vi "Dresden R2R Sputter 03.02.2018 IY24.vi"() -> ()   [LabVIEW 2009] (continued)
            n8061 = Boolean Array To Number(Boolean array=w12724) -> (number=w12730:u32)
            n8062 = Mantissa & Exponent(0:w12730) -> (2:w12723:dbl)  [unwired: 1 out]
            n8063 = case shown="0, Default" w12723 {
              tunnel: [u16 0 ("Starting Address") u16 1184 ("Starting Address") u16 1185 ("Starting Address") u16 1186 ("Starting Address") u16 1187 ("Starting Address")] -> w12720
              tunnel: [u16 0 ("Ao_1_3") "Ch4_Ao_1_0 4" "Ch4_Ao_1_1 4" "Ch4_Ao_1_2 4" "Ch4_Ao_1_3 4"] -> w12722
              frame #0 {
              }
              frame #1 {
              }
              frame #2 {
              }
              frame #3 {
              }
              frame #4 {
              }
            }
            n8064 = Build Array(w12722) -> (w12721:u16[])
            n8065 = call-poly <vilib>:"MB Serial Master Query (poly).vi"("VISA resource name"=w12719, "Starting Address"=w12720, "Registers"=w12721, "error in"=w12718, "Serial Parameters"=T39 {"Mode"=enum."RTU", "Slave Address"=6}) -> ("VISA resource name out"=w12732:refnum<visa-resource-name>, "error out"=w12731:errorcluster)  [unwired: 1 in, 12 out]
          }
          frame #7 {
            n8066 = Wait (ms)(milliseconds to wait=w12744) -> ()  [unwired: 1 out]
          }
        }
      }
      frame #1 {
        n8067 = local read "Fail_moxa4_digital3"() -> (w12747:bool)
        n8068 = local read "Fail_moxa4_digital4"() -> (w12746:bool)
        n8069 = local read "Fail_moxa4_digital1"() -> (w12745:bool)
        n8070 = local read "Fail_moxa4_digital2"() -> (w12748:bool)
        n8071 = case shown="True" w12748 {
          frame #0 {
            n8072 = local read "Ch4_Trns_gv_bp_do"() -> (w12767:bool)
            n8073 = local read "Ch4_Trns_gv_bp_di"() -> (w12766:bool)
            n8074 = Exclusive Or(1:w12767, 2:w12766) -> (0:w12765:bool)
            n8075 = feedback #213() -> (w12764:bool)  [unwired: 1 in]
            n8076 = case shown="True" w12765 {
              tunnel: [TRUE FALSE] -> w12763
              tunnel: w12764 -> [_ w12787]
              tunnel: [FALSE w12784] -> w12762
              frame #0 {
              }
              frame #1 {
                n8077 = call "Elapsed Time117"("Reset"=w12787) -> ("Elapsed Time (s)"=w12786:dbl)  [unwired: 11 in, 7 out]
                n8078 = Greater?(x=w12786, y=5.0) -> (0:w12784:bool)
              }
            }
            n8079 = local write "Trns_gv_bp_ch4_fail_top"(w12762) -> ()
            n8080 = local write "Trns_gv_bp_fail_ch4_front"(w12762) -> ()
            n8081 = local write "Ch4_Trns_gv_bp_fail"(w12762) -> ()
            n8082 = local read "Ch4_Sov_Ar_do"() -> (w12761:bool)
            n8083 = local read "Ch4_Sov_Ar_di"() -> (w12760:bool)
            n8084 = Exclusive Or(1:w12761, 2:w12760) -> (0:w12759:bool)
            n8085 = feedback #214() -> (w12758:bool)  [unwired: 1 in]
            n8086 = case shown="True" w12759 {
              tunnel: [TRUE FALSE] -> w12757
              tunnel: w12758 -> [_ w12780]
              tunnel: [FALSE w12777] -> w12756
              frame #0 {
              }
              frame #1 {
                n8087 = call "Elapsed Time110"("Reset"=w12780) -> ("Elapsed Time (s)"=w12779:dbl)  [unwired: 11 in, 7 out]
                n8088 = Greater?(x=w12779, y=5.0) -> (0:w12777:bool)
              }
            }
            n8089 = local write "ch4_sov_Ar_fail_top"(w12756) -> ()
            n8090 = local read "Ch4_Cst_fix_down_di"() -> (w12752:bool)
            n8091 = local read "Ch4_Cst_fix_do"() -> (w12751:bool)
            n8092 = Exclusive Or(1:w12752, 2:w12751) -> (0:w12755:bool)
            n8093 = feedback #215() -> (w12753:bool)  [unwired: 1 in]
            n8094 = case shown="True" w12755 {
              tunnel: [TRUE FALSE] -> w12754
              tunnel: w12753 -> [_ w12773]
              tunnel: [FALSE w12770] -> w12750
              frame #0 {
              }
              frame #1 {
                n8095 = call "Elapsed Time189"("Reset"=w12773) -> ("Elapsed Time (s)"=w12772:dbl)  [unwired: 11 in, 7 out]
                n8096 = Greater?(x=w12772, y=60.0) -> (0:w12770:bool)
              }
            }
            n8097 = local write "chamber 4 top piston failed"(w12750) -> ()
          }
          frame #1 {
            w12789 = TRUE ("Ch_bv_fail(ch4)L")
            n8098 = local write "Trns_gv_bp_ch4_fail_top"(w12789) -> ()
            n8099 = local write "Trns_gv_bp_fail_ch4_front"(w12789) -> ()
            n8100 = local write "Ch4_Trns_gv_bp_fail"(w12789) -> ()
            n8101 = local write "chamber 4 top piston failed"(w12789) -> ()
            n8102 = local write "ch4_sov_Ar_fail_top"(w12789) -> ()
          }
        }
        n8103 = case shown="True" w12745 {
          frame #0 {
            w12790 = TRUE
            n8104 = local write "ch4_atm_fail_top"(w12790) -> ()
            n8105 = local write "Ch4_Ch_vbv_fail"(w12790) -> ()
            n8106 = local write "Ch4_Ch_atm_fail"(w12790) -> ()
            n8107 = local write "ch1_bg_bv_fail_top"(w12790) -> ()
            n8108 = local write "Ch4_Bg_bv_fail"(w12790) -> ()
            n8109 = local write "Ch4_Tp_bv_fail"(w12790) -> ()
            n8110 = local write "Ch4_Mp_fail"(w12790) -> ()
            n8111 = local write "ch4_bg_bv_fail_top"(w12790) -> ()
            n8112 = local write "Ch4_Ch_cc_fail"(w12790) -> ()
            n8113 = local write "Ch4_Pl_vbv_fail"(w12790) -> ()
            n8114 = local write "Ch4_Pl_atm_fail"(w12790) -> ()
            n8115 = local write "ch4_cc_fail_top"(w12790) -> ()
          }
          frame #1 {
            n8116 = local read "Ch4_Mp_do"() -> (w12807:bool)
            n8117 = local read "Ch4_Mp_di"() -> (w12808:bool)
            n8118 = Exclusive Or(1:w12807, 2:w12808) -> (0:w12824:bool)
            n8119 = feedback #216() -> (w12825:bool)  [unwired: 1 in]
            n8120 = case shown="True" w12824 {
              tunnel: [TRUE FALSE] -> w12826
              tunnel: w12825 -> [_ w12867]
              tunnel: [FALSE w12864] -> w12806
              frame #0 {
              }
              frame #1 {
                n8121 = call "Elapsed Time122"("Reset"=w12867) -> ("Elapsed Time (s)"=w12866:dbl)  [unwired: 11 in, 7 out]
                n8122 = Greater?(x=w12866, y=5.0) -> (0:w12864:bool)
              }
            }
            n8123 = local write "Ch4_Mp_fail"(w12806) -> ()
            n8124 = local read "Ch4_Tp_bv_do"() -> (w12804:bool)
            n8125 = local read "Ch4_Tp_bv_di"() -> (w12805:bool)
            n8126 = Exclusive Or(1:w12804, 2:w12805) -> (0:w12823:bool)
            n8127 = feedback #217() -> (w12822:bool)  [unwired: 1 in]
            n8128 = case shown="True" w12823 {
              tunnel: [TRUE FALSE] -> w12821
              tunnel: w12822 -> [_ w12860]
              tunnel: [FALSE w12857] -> w12803
              frame #0 {
              }
              frame #1 {
                n8129 = call "Elapsed Time123"("Reset"=w12860) -> ("Elapsed Time (s)"=w12859:dbl)  [unwired: 11 in, 7 out]
                n8130 = Greater?(x=w12859, y=5.0) -> (0:w12857:bool)
              }
            }
            n8131 = local write "Ch4_Tp_bv_fail"(w12803) -> ()
            n8132 = local read "Ch4_Bg_bv_di"() -> (w12802:bool)
            n8133 = local read "Ch4_Bg_bv_do"() -> (w12801:bool)
            n8134 = Exclusive Or(1:w12801, 2:w12802) -> (0:w12818:bool)
            n8135 = feedback #218() -> (w12819:bool)  [unwired: 1 in]
            n8136 = case shown="True" w12818 {
              tunnel: [TRUE FALSE] -> w12820
              tunnel: w12819 -> [_ w12853]
              tunnel: [FALSE w12850] -> w12792
              frame #0 {
              }
              frame #1 {
                n8137 = call "Elapsed Time124"("Reset"=w12853) -> ("Elapsed Time (s)"=w12852:dbl)  [unwired: 11 in, 7 out]
                n8138 = Greater?(x=w12852, y=5.0) -> (0:w12850:bool)
              }
            }
            n8139 = local write "ch4_bg_bv_fail_top"(w12792) -> ()
            n8140 = local write "Ch4_Bg_bv_fail"(w12792) -> ()
            n8141 = local read "Ch4_Ch_vbv_do"() -> (w12799:bool)
            n8142 = local read "Ch4_Ch_vbv_di"() -> (w12800:bool)
            n8143 = Exclusive Or(1:w12799, 2:w12800) -> (0:w12817:bool)
            n8144 = feedback #219() -> (w12816:bool)  [unwired: 1 in]
            n8145 = case shown="True" w12817 {
              tunnel: [TRUE FALSE] -> w12815
              tunnel: w12816 -> [_ w12846]
              tunnel: [FALSE w12843] -> w12793
              frame #0 {
              }
              frame #1 {
                n8146 = call "Elapsed Time125"("Reset"=w12846) -> ("Elapsed Time (s)"=w12845:dbl)  [unwired: 11 in, 7 out]
                n8147 = Greater?(x=w12845, y=5.0) -> (0:w12843:bool)
              }
            }
            n8148 = local write "Ch4_Ch_vbv_fail"(w12793) -> ()
            n8149 = local read "Ch4_Pl_vbv_do"() -> (w12796:bool)
            n8150 = local read "Ch4_Pl_vbv_di"() -> (w12797:bool)
            n8151 = Exclusive Or(1:w12796, 2:w12797) -> (0:w12814:bool)
            n8152 = feedback #220() -> (w12813:bool)  [unwired: 1 in]
            n8153 = case shown="True" w12814 {
              tunnel: [TRUE FALSE] -> w12812
              tunnel: w12813 -> [_ w12839]
              tunnel: [FALSE w12836] -> w12798
              frame #0 {
              }
              frame #1 {
                n8154 = call "Elapsed Time127"("Reset"=w12839) -> ("Elapsed Time (s)"=w12838:dbl)  [unwired: 11 in, 7 out]
                n8155 = Greater?(x=w12838, y=5.0) -> (0:w12836:bool)
              }
            }
            n8156 = local write "Ch4_Pl_vbv_fail"(w12798) -> ()
            n8157 = local read "Ch4_Cc_on_off_di"() -> (w12795:bool)
            n8158 = local read "Ch4_Cc_on_off_do"() -> (w12794:bool)
            n8159 = feedback #221() -> (w12810:bool)  [unwired: 1 in]
            n8160 = Exclusive Or(1:w12794, 2:w12795) -> (0:w12811:bool)
            n8161 = case shown="True" w12811 {
              tunnel: [TRUE FALSE] -> w12809
              tunnel: w12810 -> [_ w12832]
              tunnel: [FALSE w12829] -> w12791
              frame #0 {
              }
              frame #1 {
                n8162 = call "Elapsed Time129"("Reset"=w12832) -> ("Elapsed Time (s)"=w12831:dbl)  [unwired: 11 in, 7 out]
                n8163 = Greater?(x=w12831, y=5.0) -> (0:w12829:bool)
              }
            }
            n8164 = local write "ch4_cc_fail_top"(w12791) -> ()
          }
        }
        n8165 = case shown="True" w12747 {
          frame #0 {
          }
          frame #1 {
          }
        }
        n8166 = case shown="False" w12746 {
          frame #0 {
          }
          frame #1 {
            n8167 = local write "Ch4_Trns_gv_bp_fail"(TRUE ("Ch_bv_fail(ch4)L")) -> ()
          }
        }
      }
    }
    n8168 = Wait Until Next ms Multiple(millisecond multiple=u32 300) -> ()  [unwired: 1 out]
  }
  n8169 = while {
    tunnel: w760 -> [w12875]
    tunnel: [w12874] -> w744
    tunnel: [w12873] -> w759
    tunnel: w761 -> [w12872]
    tunnel: "milliseconds to wait 4" -> [w12870]
    stop <- FALSE stop-if-true
    n8170 = Wait Until Next ms Multiple(millisecond multiple=u32 300) -> ()  [unwired: 1 out]
    n8171 = stacked-sequence {
      tunnel: w12875 -> [w12880 _]
      tunnel: [w12879 _] -> w12874
      tunnel: [w12877 _] -> w12873
      tunnel: w12872 -> [w12878 _]
      tunnel: w12870 -> [w12876 _]
      frame #0 {
        n8172 = stacked-sequence {
          tunnel: w12878 -> [w12903 _ _ _ _ _ _ _ _ _]
          tunnel: w12880 -> [w12902 _ _ _ _ _ _ _ _ _]
          tunnel: [_ _ _ _ _ _ _ _ w13238 _] -> w12879
          tunnel: [_ _ _ _ _ _ _ _ w13237 _] -> w12877
          tunnel: w12876 -> [_ w12973 _ w12993 _ w13048 _ w13224 _ w13257]
          frame #0 {
            # "Digital I/O & Analog \nOutput Part"
            n8173 = call-poly <vilib>:"MB Serial Master Query (poly).vi"("VISA resource name"=w12903, "Starting Address"=u16 0, "Quantity"=u16 8, "error in"=w12902, "Serial Parameters"=T39 {"Mode"=enum."RTU", "Slave Address"=1}) -> ("VISA resource name out"=w12901:refnum<visa-resource-name>, "Discrete Inputs"=w12962:bool[], "error out"=w12900:errorcluster)  [unwired: 1 in, 11 out]
            n8174 = Index Array(array=w12962, index=6) -> (element=w12957:bool)
            "Ch3_Pl_atm_di" <- w12957
            n8175 = Index Array(array=w12962, index=7) -> (element=w12886:bool)
            "Ch3_Cc_on_off_di" <- w12886
            n8176 = Index Array(array=w12962, index=5) -> (element=w12891:bool)
            "Ch3_Pl_vbv_di" <- w12891
            n8177 = Index Array(array=w12962, index=0) -> (element=w12960:bool)
            "Ch3_Mp_di" <- w12960
            n8178 = Index Array(array=w12962, index=1) -> (element=w12959:bool)
            "Ch3_Tp_bv_di" <- w12959
            n8179 = Index Array(array=w12962, index=2) -> (element=w12888:bool)
            "Ch3_Bg_bv_di" <- w12888
            n8180 = Index Array(array=w12962, index=3) -> (element=w12958:bool)
            "Ch3_Ch_vbv_di" <- w12958
            n8181 = Index Array(array=w12962, index=4) -> (element=w12887:bool)
            "Ch3_Ch_atm_di" <- w12887
            n8182 = local write "Ch3_Mp_on"(w12960) -> ()
            n8183 = local write "Ch3_Tp_bv_on"(w12959) -> ()
            n8184 = local write "ch3_bg_bv_on_top"(w12888) -> ()
            n8185 = local write "Ch3_Bg_bv_on"(w12888) -> ()
            n8186 = local write "Ch3_Ch_vbv_on"(w12958) -> ()
            n8187 = local write "ch3_atm_on_top"(w12887) -> ()
            n8188 = local write "Ch3_Ch_atm_on"(w12887) -> ()
            n8189 = local write "Ch3_Pl_vbv_on"(w12891) -> ()
            n8190 = local write "Ch3_Pl_atm_on"(w12957) -> ()
            n8191 = local write "Ch3_Ch_cc_on"(w12886) -> ()
            n8192 = local write "ch3_cc_on_top"(w12886) -> ()
            n8193 = local read "Load_dido"() -> (w12890:bool)
            n8194 = case shown="True" w12890 {
              frame #0 {
              }
              frame #1 {
                n8195 = Wait (ms)(milliseconds to wait=u32 2000) -> ()  [unwired: 1 out]
              }
            }
            n8196 = call-poly <vilib>:"MB Serial Master Query (poly).vi"("VISA resource name"=w12901, "Starting Address"=u16 0, "Quantity"=u16 8, "error in"=w12900, "Serial Parameters"=T39 {"Mode"=enum."RTU", "Slave Address"=2}) -> ("VISA resource name out"=w12899:refnum<visa-resource-name>, "Discrete Inputs"=w12947:bool[], "error out"=w12898:errorcluster)  [unwired: 1 in, 11 out]
            n8197 = Index Array(array=w12947, index=2) -> (element=→"Ch3_Trns_gv_close_di":bool)
            n8198 = Index Array(array=w12947, index=0) -> (element=w12889:bool)
            "Ch3_Sov_Ar_di" <- w12889
            n8199 = Index Array(array=w12947, index=1) -> (element=w12883:bool)
            "Ch3_Trns_gv_open_di" <- w12883
            n8200 = Index Array(array=w12947, index=5) -> (element=w12884:bool)
            "Ch3_Cst_fix_down_di" <- w12884
            n8201 = Index Array(array=w12947, index=6) -> (element=→"Ch3_Pet_cool_up_di":bool)
            n8202 = Index Array(array=w12947, index=7) -> (element=→"Ch3_Pet_cool_down_di":bool)
            n8203 = Index Array(array=w12947, index=3) -> (element=w12881:bool)
            "Ch3_Trns_gv_bp_di" <- w12881
            n8204 = Index Array(array=w12947, index=4) -> (element=→"Ch3_Cst_fix_up_di":bool)
            n8205 = local write "Ch3_trns_gv_bp_on_front"(w12881) -> ()
            n8206 = local write "gv front_open_ch3_4"(w12883) -> ()
            n8207 = local write "Trns_gv_3_4_on"(w12883) -> ()
            n8208 = local write "gv top open_ch3_4"(w12883) -> ()
            n8209 = local write "gv front open ch4_3"(w12883) -> ()
            n8210 = local write "gv top open ch_4_3"(w12883) -> ()
            n8211 = local write "Ch3_Trns_gv_bp_on"(w12881) -> ()
            n8212 = local write "ch3_sov_Ar_on_top"(w12889) -> ()
            n8213 = local write "chamber 3 top piston open"(w12884) -> ()
            n8214 = local write "ch3_trns_gv_bp_on_top"(w12881) -> ()
            n8215 = call-poly <vilib>:"MB Serial Master Query (poly).vi"("VISA resource name"=w12899, "Starting Address"=u16 0, "Quantity"=u16 8, "error in"=w12898, "Serial Parameters"=T39 {"Mode"=enum."RTU", "Slave Address"=3}) -> ("VISA resource name out"=w12897:refnum<visa-resource-name>, "Discrete Inputs"=w12907:bool[], "error out"=w12896:errorcluster)  [unwired: 1 in, 11 out]
            n8216 = Index Array(array=w12907, index=5) -> (element=→"Ch3_SRV2_counter_di":bool)
            n8217 = Index Array(array=w12907, index=6) -> (element=→"Ch3_WFS_di":bool)
            n8218 = Index Array(array=w12907, index=7) -> (element=w12882:bool)
            "Ch3_Trns_gv_bp2_di" <- w12882
            n8219 = Index Array(array=w12907, index=0) -> (element=→"Ch3_SRV1_PIST For_di":bool)
            n8220 = Index Array(array=w12907, index=1) -> (element=→"Ch3_SRV1_PIST_Back_di":bool)
            n8221 = Index Array(array=w12907, index=2) -> (element=→"Ch3_SRV_start_stop_di":bool)
            n8222 = Index Array(array=w12907, index=3) -> (element=→"Ch3_SRV_left_direction_di":bool)
            n8223 = Index Array(array=w12907, index=4) -> (element=→"Ch3_SRV1_counter_di":bool)
            n8224 = local write "Ch3_Trns_gv_bp2_on"(w12882) -> ()
            n8225 = local write "ch3_trns_gv_bp2_on_top"(w12882) -> ()
            n8226 = local write "Ch3_trns_gv_bp2_on_front"(w12882) -> ()
            n8227 = call-poly <vilib>:"MB Serial Master Query (poly).vi"("VISA resource name"=w12897, "Starting Address"=u16 0, "Quantity"=u16 8, "error in"=w12896, "Serial Parameters"=T39 {"Mode"=enum."RTU", "Slave Address"=4}) -> ("VISA resource name out"=w12895:refnum<visa-resource-name>, "Discrete Inputs"=w12931:bool[], "error out"=w12894:errorcluster)  [unwired: 1 in, 11 out]
            n8228 = Index Array(array=w12931, index=5) -> (element=→"Ch3_Right_slow_di":bool)
            n8229 = Index Array(array=w12931, index=6) -> (element=→"Ch3_Left_slow_di":bool)
            n8230 = Index Array(array=w12931, index=7) -> (element=→"Ch3_Left_limit_di":bool)
            n8231 = Index Array(array=w12931, index=0) -> (element=→"Ch3_Air_press_di":bool)
            n8232 = Index Array(array=w12931, index=1) -> (element=→"Ch3_Ds_di":bool)
            n8233 = Index Array(array=w12931, index=2) -> (element=→"Ch3_TGV_control_di":bool)
            n8234 = Index Array(array=w12931, index=3) -> (element=→"Ch3_Trns_interlock_di":bool)
            n8235 = Index Array(array=w12931, index=4) -> (element=→"Ch3_Right_limit_di":bool)
          }
          frame #1 {
            n8236 = Wait (ms)(milliseconds to wait=w12973) -> ()  [unwired: 1 out]
          }
          frame #2 {
            n8237 = local read "Load_dido"() -> (w12974:bool)
            n8238 = case shown="True" w12974 {
              frame #0 {
              }
              frame #1 {
                n8239 = while {
                  stop <- w12986 stop-if-true
                  n8240 = local read "Ch3_Mp_di"() -> (w12992:bool)
                  n8241 = local read "Ch3_Tp_bv_di"() -> (w12991:bool)
                  n8242 = local read "Ch3_Bg_bv_di"() -> (w12990:bool)
                  n8243 = local read "Ch3_Ch_vbv_di"() -> (w12989:bool)
                  n8244 = local read "Ch3_Pl_vbv_di"() -> (w12988:bool)
                  n8245 = local read "Ch3_Cc_on_off_di"() -> (w12987:bool)
                  n8246 = local write "Ch3_Mp_do"(w12992) -> ()
                  n8247 = local write "Ch3_Tp_bv_do"(w12991) -> ()
                  n8248 = local write "Ch3_Bg_bv_do"(w12990) -> ()
                  n8249 = local write "Ch3_Ch_vbv_do"(w12989) -> ()
                  n8250 = local write "Ch3_Pl_vbv_do"(w12988) -> ()
                  n8251 = local write "Ch3_Cc_on_off_do"(w12987) -> ()
                  n8252 = local read "Ch3_Trns_gv_bp2_di"() -> (w12982:bool)
                  n8253 = Wait Until Next ms Multiple(millisecond multiple=u32 300) -> ()  [unwired: 1 out]
                  n8254 = local read "Ch3_WFS_di"() -> (w12983:bool)
                  n8255 = local write "Ch3_WFC_do"(w12983) -> ()
                  n8256 = local write "Ch3_Trns_gv_bp2_do"(w12982) -> ()
                  n8257 = local read "Ch3_Cst_fix_down_di"() -> (w12977:bool)
                  n8258 = local read "Ch3_Sov_Ar_di"() -> (w12981:bool)
                  n8259 = local read "Ch3_Trns_gv_open_di"() -> (w12980:bool)
                  n8260 = local read "Ch3_Trns_gv_close_di"() -> (w12979:bool)
                  n8261 = local read "Ch3_Pet_cool_up_di"() -> (w12976:bool)
                  n8262 = local read "Ch3_Pet_cool_down_di"() -> (w12975:bool)
                  n8263 = local read "Ch3_Trns_gv_bp_di"() -> (w12978:bool)
                  n8264 = local write "Ch3_Sov_Ar_do"(w12981) -> ()
                  n8265 = local write "Ch3_Trns_gv_open_do"(w12980) -> ()
                  n8266 = local write "Ch3_Trns_gv_close_do"(w12979) -> ()
                  n8267 = local write "Ch3_Pet_cool_up_do"(w12976) -> ()
                  n8268 = local write "Ch3_Pet_cool_down_do"(w12975) -> ()
                  n8269 = local write "Ch3_Trns_gv_bp_do"(w12978) -> ()
                  n8270 = local write "Ch3_Cst_fix_do"(w12977) -> ()
                  n8271 = local read "Load_dido"() -> (w12985:bool)
                  n8272 = Not(x=w12985) -> (.not. x?=w12986:bool)
                }
              }
            }
          }
          frame #3 {
            n8273 = Wait (ms)(milliseconds to wait=w12993) -> ()  [unwired: 1 out]
          }
          frame #4 {
            n8274 = Build Array("Ch3_Mp_do", "Ch3_Tp_bv_do", "Ch3_Bg_bv_do", "Ch3_Ch_vbv_do", "Ch3_Ch_atm_do", "Ch3_Pl_vbv_do", "Ch3_Pl_atm_do", "Ch3_Cc_on_off_do") -> (w13018:bool[])
            n8275 = call-poly <vilib>:"MB Serial Master Query (poly).vi"("VISA resource name"=w13005, "Starting Address"=u16 320, "Coils"=w13018, "error in"=w13004, "Serial Parameters"=T39 {"Mode"=enum."RTU", "Slave Address"=1}) -> ("VISA resource name out"=w13003:refnum<visa-resource-name>, "error out"=w13002:errorcluster)  [unwired: 1 in, 12 out]
            n8276 = Build Array("Ch3_Sov_Ar_do", "Ch3_Trns_gv_open_do", "Ch3_Trns_gv_close_do", "Ch3_Trns_gv_bp_do", "Ch3_Cst_fix_do", "Ch3_2_5_do", "Ch3_Pet_cool_up_do", "Ch3_Pet_cool_down_do") -> (w13028:bool[])
            n8277 = call-poly <vilib>:"MB Serial Master Query (poly).vi"("VISA resource name"=w13003, "Starting Address"=u16 320, "Coils"=w13028, "error in"=w13002, "Serial Parameters"=T39 {"Mode"=enum."RTU", "Slave Address"=2}) -> ("VISA resource name out"=w13001:refnum<visa-resource-name>, "error out"=w13000:errorcluster)  [unwired: 1 in, 12 out]
            n8278 = Build Array("Ch3_SRV1_PIST For_do", "Ch3_SRV1_PIST_Back_do", "Ch3_SRV_start_stop_do", "Ch3_SRV_counterclockwise_direction_do", "Ch3_Do_3_4", "Ch3_Do_3_5", "Ch3_WFC_do", "Ch3_Trns_gv_bp2_do") -> (w13036:bool[])
            n8279 = call-poly <vilib>:"MB Serial Master Query (poly).vi"("VISA resource name"=w13001, "Starting Address"=u16 320, "Coils"=w13036, "error in"=w13000, "Serial Parameters"=T39 {"Mode"=enum."RTU", "Slave Address"=3}) -> ("VISA resource name out"=w12998:refnum<visa-resource-name>, "error out"=w12999:errorcluster)  [unwired: 1 in, 12 out]
            n8280 = Build Array("Ch3_4_0_do", "Ch3_4_1_do", "Ch3_TGV_control_do", "Ch3_4_3_do", "Ch3_4_4_do", "Ch3_Do_4_5_do", "Ch3_Do_4_6_do", "Ch3_Do_4_6_do") -> (w13038:bool[])
            n8281 = call-poly <vilib>:"MB Serial Master Query (poly).vi"("VISA resource name"=w12998, "Starting Address"=u16 320, "Coils"=w13038, "error in"=w12999, "Serial Parameters"=T39 {"Mode"=enum."RTU", "Slave Address"=4}) -> ("VISA resource name out"=w12997:refnum<visa-resource-name>, "error out"=w12996:errorcluster)  [unwired: 1 in, 12 out]
          }
          frame #5 {
            n8282 = Wait (ms)(milliseconds to wait=w13048) -> ()  [unwired: 1 out]
          }
          frame #6 {
            n8283 = local read "1bit="() -> (w13059:dbl)
            n8284 = local read "1bit="() -> (w13061:dbl)
            n8285 = local read "1bit="() -> (w13053:dbl)
            n8286 = call-poly <vilib>:"MB Serial Master Query (poly).vi"("VISA resource name"=w13057, "Starting Address"=u16 704, "Quantity"=u16 8, "error in"=w13055, "Serial Parameters"=T39 {"Mode"=enum."RTU", "Slave Address"=5}) -> ("VISA resource name out"=w13056:refnum<visa-resource-name>, "Input Registers"=w13069:u16[], "error out"=w13054:errorcluster)  [unwired: 1 in, 11 out]
            n8287 = Index Array(array=w13069, index=5) -> (element=→"Ch1_Ai_1_5 3":u16)
            n8288 = Index Array(array=w13069, index=6) -> (element=→"Ch1_Ai_1_6 3":u16)
            n8289 = Index Array(array=w13069, index=7) -> (element=→"Ch1_Ai_1_7 3":u16)
            n8290 = Index Array(array=w13069, index=0) -> (element=w13063:u16)
            "Ch3_Ai_PL_PG" <- w13063
            n8291 = Index Array(array=w13069, index=1) -> (element=w13049:u16)
            "Ch3_Ai_CH_PG" <- w13049
            n8292 = Multiply(x=w13061, y=w13049) -> (x*y=w13060:dbl)
            n8293 = stacked-sequence {
              tunnel: w13060 -> [w13161]
              frame #0 {
                # "CH-PG 0-10 Volt okuma"
                n8294 = feedback #222() -> (w13172:dbl)  [unwired: 1 in]
                n8295 = feedback #223() -> (w13170:dbl)  [unwired: 1 in]
                n8296 = feedback #224() -> (w13169:dbl)  [unwired: 1 in]
                n8297 = feedback #225() -> (w13168:dbl)  [unwired: 1 in]
                n8298 = feedback #226() -> (w13167:dbl)  [unwired: 1 in]
                n8299 = feedback #227() -> (w13166:dbl)  [unwired: 1 in]
                n8300 = feedback #228() -> (w13165:dbl)  [unwired: 1 in]
                n8301 = feedback #229() -> (w13163:dbl)  [unwired: 1 in]
                n8302 = feedback #230() -> (w13164:dbl)  [unwired: 1 in]
                n8303 = Compound Arithmetic op=ADD(w13161, w13172, w13170, w13169, w13168, w13167, w13166, w13165, w13163, w13164) -> (w13171:dbl)
                n8304 = local read "Ch_pg_volt_instantaneos_ch3"() -> (w13155:u16)
                n8305 = Divide(x=w13171, y=u16 10) -> (x/y=w13156:dbl)
                "Ch_pg_volt_ch3" <- w13156
                n8306 = Greater Or Equal?(x=w13155, y=u16 1) -> (x >= y?=w13154:bool)
                n8307 = feedback #231() -> (w13159:bool)  [unwired: 1 in]
                n8308 = case shown="True" w13154 {
                  tunnel: w13156 -> [_ w13184]
                  tunnel: [FALSE TRUE] -> w13158
                  tunnel: w13159 -> [w13175 _]
                  tunnel: [w13174 FALSE ("Bg_gui")] -> w13160
                  frame #0 {
                    n8309 = local write "Ch3_Ch_pg_on"(FALSE ("Bg_gui")) -> ()
                    n8310 = call "Elapsed Time143"("Reset"=w13175) -> ("Elapsed Time (s)"=w13178:dbl)  [unwired: 11 in, 7 out]
                    n8311 = Greater Or Equal?(x=w13178, y=3.0) -> (x >= y?=w13174:bool)
                  }
                  frame #1 {
                    n8312 = Subtract(x=w13184, y=5.625) -> (x-y=w13186:dbl)
                    n8313 = Power Of 10(x=w13186) -> (10^x=w13185:dbl)
                    n8314 = In Range and Coerce(upper limit=760.0, x=w13185, lower limit=0.000375) -> (coerced(x)=→"Ch_pg_press_ch3" →"Ch_pg_press_ch3_gui":dbl)  [unwired: 1 out]
                    n8315 = local write "Ch3_Ch_pg_on"(TRUE ("Bg_gui")) -> ()
                  }
                }
                n8316 = local write "Ch3_Ch_pg_fail"(w13160) -> ()
                "Ch_pg_volt_instantaneos_ch3" <- w13161
              }
            }
            n8317 = Index Array(array=w13069, index=2) -> (element=w13050:u16)
            "Ch3_Ai_CH-CC" <- w13050
            n8318 = Multiply(x=w13059, y=w13050) -> (x*y=w13058:dbl)
            n8319 = stacked-sequence {
              tunnel: w13058 -> [w13106]
              frame #0 {
                # "CH-CC 0-10 Volt okuma"
                n8320 = feedback #232() -> (w13115:dbl)  [unwired: 1 in]
                n8321 = feedback #233() -> (w13116:dbl)  [unwired: 1 in]
                n8322 = feedback #234() -> (w13117:dbl)  [unwired: 1 in]
                n8323 = feedback #235() -> (w13118:dbl)  [unwired: 1 in]
                n8324 = feedback #236() -> (w13119:dbl)  [unwired: 1 in]
                n8325 = feedback #237() -> (w13120:dbl)  [unwired: 1 in]
                n8326 = feedback #238() -> (w13121:dbl)  [unwired: 1 in]
                n8327 = feedback #239() -> (w13133:dbl)  [unwired: 1 in]
                n8328 = feedback #240() -> (w13122:dbl)  [unwired: 1 in]
                n8329 = feedback #241() -> (w13123:dbl)  [unwired: 1 in]
                n8330 = feedback #242() -> (w13124:dbl)  [unwired: 1 in]
                n8331 = feedback #243() -> (w13125:dbl)  [unwired: 1 in]
                n8332 = feedback #244() -> (w13126:dbl)  [unwired: 1 in]
                n8333 = feedback #245() -> (w13127:dbl)  [unwired: 1 in]
                n8334 = feedback #246() -> (w13128:dbl)  [unwired: 1 in]
                n8335 = feedback #247() -> (w13129:dbl)  [unwired: 1 in]
                n8336 = feedback #248() -> (w13130:dbl)  [unwired: 1 in]
                n8337 = feedback #249() -> (w13131:dbl)  [unwired: 1 in]
                n8338 = feedback #250() -> (w13132:dbl)  [unwired: 1 in]
                n8339 = Compound Arithmetic op=ADD(w13106, w13115, w13116, w13117, w13118, w13119, w13120, w13121, w13133, w13122, w13123, w13124, w13125, w13126, w13127, w13128, w13129, w13130, w13131, w13132) -> (w13114:dbl)
                n8340 = Divide(x=w13114, y=u16 20) -> (x/y=w13110:dbl)
                "Ch_CC_volt ch3" <- w13110
                n8341 = feedback #251() -> (w13107:bool)  [unwired: 1 in]
                n8342 = Greater?(x=w13110, y=1.0) -> (0:w13111:bool)
                n8343 = case shown="True" w13111 {
                  tunnel: w13110 -> [_ w13150]
                  tunnel: [w13141 FALSE] -> w13109
                  tunnel: [FALSE ("Ch_cc_on(ch1)") TRUE] -> w13108
                  tunnel: w13107 -> [_ _]
                  frame #0 {
                    n8344 = local read "Ch3_Cc_on_off_di"() -> (w13135:bool)
                    n8345 = call "Elapsed Time87"() -> ("Elapsed Time (s)"=w13144:dbl)  [unwired: 12 in, 7 out]
                    n8346 = Not(x=w13135) -> (.not. x?=w13138:bool)
                    n8347 = Greater Or Equal?(x=w13144, y=3.0) -> (x >= y?=w13143:bool)
                    n8348 = call "Elapsed Time88"("Reset"=w13138) -> ("Elapsed Time (s)"=w13140:dbl)  [unwired: 11 in, 7 out]
                    n8349 = local write "Ch3_Ch_cc_on"(FALSE ("Ch_cc_on(ch1)")) -> ()
                    n8350 = Greater Or Equal?(x=w13140, y=3.0) -> (x >= y?=w13137:bool)
                    n8351 = And(x=w13143, y=w13137) -> (x .and. y?=w13141:bool)
                  }
                  frame #1 {
                    n8352 = Subtract(x=w13150, y=10.625) -> (x-y=w13147:dbl)
                    n8353 = Power Of 10(x=w13147) -> (10^x=w13146:dbl)
                    n8354 = In Range and Coerce(upper limit=0.0075, x=w13146, lower limit=1.5e-09) -> (coerced(x)=→"Ch_CC_press_ch3" →"Ch_CC_press_ch3 2":dbl)  [unwired: 1 out]
                  }
                }
                n8355 = local write "Ch3_Ch_cc_fail"(w13109) -> ()
                "Ch_CC_volt_instantaneos_ch3" <- w13106
              }
            }
            n8356 = Index Array(array=w13069, index=3) -> (element=w13051:u16)
            "Ch3_Ai_MFC_Ar_2" <- w13051
            n8357 = Multiply(x=w13053, y=w13051) -> (x*y=w13052:dbl)
            n8358 = stacked-sequence {
              tunnel: w13052 -> [w13082]
              frame #0 {
                # "MFC AR 0-5 volt okuma"
                n8359 = feedback #252() -> (w13087:dbl)  [unwired: 1 in]
                n8360 = feedback #253() -> (w13088:dbl)  [unwired: 1 in]
                n8361 = feedback #254() -> (w13089:dbl)  [unwired: 1 in]
                n8362 = feedback #255() -> (w13090:dbl)  [unwired: 1 in]
                n8363 = Compound Arithmetic op=ADD(w13082, w13087, w13088, w13089, w13090) -> (w13086:dbl)
                n8364 = Divide(x=w13086, y=u16 5) -> (x/y=w13081:dbl)
                "MFC_volt 2" <- w13081
                n8365 = Greater?(x=w13081, y=0.1) -> (0:w13083:bool)
                n8366 = case shown="False" w13083 {
                  tunnel: w13081 -> [_ w13094]
                  frame #0 {
                    w13091 = 0.0 ("Ar_sccm_act 2")
                    n8367 = local write "Ar_sccm_act 2"(w13091) -> ()
                    n8368 = local write "Ar_sccm_act gui 2"(w13091) -> ()
                    n8369 = local write "Ar_sccm_act 4"(w13091) -> ()
                  }
                  frame #1 {
                    # "200 ccm/5V\nçarpan 40"
                    n8370 = Multiply(x=w13094, y=40.0) -> (x*y=→"Ar_sccm_act 2" →"Ar_sccm_act gui 2" →"Ar_sccm_act 4":dbl)
                  }
                }
                "MFC_volt_instantaneous 2" <- w13082
              }
            }
            n8371 = Index Array(array=w13069, index=4) -> (element=→"Ch3_Ai_1_4":u16)
            n8372 = local read "1bit="() -> (w13064:dbl)
            n8373 = Multiply(x=w13064, y=w13063) -> (x*y=w13062:dbl)
            n8374 = stacked-sequence {
              tunnel: w13062 -> [w13196]
              frame #0 {
                # "PL-PG 0-10 Volt okuma"
                n8375 = feedback #256() -> (w13207:dbl)  [unwired: 1 in]
                n8376 = feedback #257() -> (w13205:dbl)  [unwired: 1 in]
                n8377 = feedback #258() -> (w13204:dbl)  [unwired: 1 in]
                n8378 = feedback #259() -> (w13203:dbl)  [unwired: 1 in]
                n8379 = feedback #260() -> (w13202:dbl)  [unwired: 1 in]
                n8380 = feedback #261() -> (w13201:dbl)  [unwired: 1 in]
                n8381 = feedback #262() -> (w13200:dbl)  [unwired: 1 in]
                n8382 = feedback #263() -> (w13198:dbl)  [unwired: 1 in]
                n8383 = feedback #264() -> (w13199:dbl)  [unwired: 1 in]
                n8384 = Compound Arithmetic op=ADD(w13196, w13207, w13205, w13204, w13203, w13202, w13201, w13200, w13198, w13199) -> (w13206:dbl)
                n8385 = local read "Pl_pg_volt_instantaneous_ch3"() -> (w13194:u16)
                n8386 = Divide(x=w13206, y=10.0) -> (x/y=w13195:dbl)
                "Pl_pg_volt_ch3" <- w13195
                n8387 = Greater Or Equal?(x=w13194, y=u16 1) -> (x >= y?=w13193:bool)
                n8388 = feedback #265() -> (w13190:bool)  [unwired: 1 in]
                n8389 = case shown="False" w13193 {
                  tunnel: w13195 -> [_ w13219]
                  tunnel: [FALSE TRUE] -> w13191
                  tunnel: w13190 -> [w13210 _]
                  tunnel: [w13209 FALSE ("Bg_gui")] -> w13189
                  frame #0 {
                    n8390 = local write "Ch3_Pl_pg_on"(FALSE ("Bg_gui")) -> ()
                    n8391 = call "Elapsed Time89"("Reset"=w13210) -> ("Elapsed Time (s)"=w13213:dbl)  [unwired: 11 in, 7 out]
                    n8392 = Greater Or Equal?(x=w13213, y=3.0) -> (x >= y?=w13209:bool)
                  }
                  frame #1 {
                    n8393 = Subtract(x=w13219, y=5.625) -> (x-y=w13221:dbl)
                    n8394 = local write "Ch3_Pl_pg_on"(TRUE ("Bg_gui")) -> ()
                    n8395 = Power Of 10(x=w13221) -> (10^x=w13220:dbl)
                    n8396 = In Range and Coerce(upper limit=760.0, x=w13220, lower limit=0.000375) -> (coerced(x)=→"Pl_pg_press_ch3" →"Pl_pg_press_ch3_gui":dbl)  [unwired: 1 out]
                  }
                }
                n8397 = local write "Ch3_Pl_pg_fail"(w13189) -> ()
                "Pl_pg_volt_instantaneous_ch3" <- w13196
              }
            }
            n8398 = stacked-sequence {
              frame #0 {
                n8399 = local read "Ch3_Cc_on_off_di"() -> (w13095:bool)
                n8400 = case shown="False" w13095 {
                  frame #0 {
                    n8401 = local read "Ch_pg_press_ch3"() -> (→"Ch3_pressure" →"Ch3_pressure2":dbl)
                  }
                  frame #1 {
                    n8402 = local read "Ch_CC_volt ch3"() -> (w13103:u16)
                    n8403 = local read "Ch_pg_volt_ch3"() -> (w13101:u16)
                    n8404 = Greater?(x=w13103, y=u16 2) -> (0:w13100:bool)
                    n8405 = Less?(x=w13101, y=u16 4) -> (x < y?=w13099:bool)
                    n8406 = Or(x=w13100, y=w13099) -> (x .or. y?=w13098:bool)
                    n8407 = case shown="True" w13098 {
                      frame #0 {
                        n8408 = local read "Ch_pg_press_ch3"() -> (w13104:dbl)
                        n8409 = local write "Ch3_pressure"(w13104) -> ()
                        n8410 = local write "Ch3_pressure2"(w13104) -> ()
                      }
                      frame #1 {
                        n8411 = local read "Ch_CC_press_ch3"() -> (w13105:dbl)
                        n8412 = local write "Ch3_pressure"(w13105) -> ()
                        n8413 = local write "Ch3_pressure2"(w13105) -> ()
                      }
                    }
                  }
                }
              }
            }
          }
          frame #7 {
            n8414 = Wait (ms)(milliseconds to wait=w13224) -> ()  [unwired: 1 out]
          }
          frame #8 {
            n8415 = Build Array(FALSE, "Ch3_Ao_1_0", "Ch3_Ao_1_1", "Ch3_Ao_1_2", "Mfc2_Ar _3_4_set") -> (w13231:bool[])
            n8416 = Boolean Array To Number(Boolean array=w13231) -> (number=w13236:u32)
            n8417 = Mantissa & Exponent(0:w13236) -> (2:w13230:dbl)  [unwired: 1 out]
            n8418 = case shown="4" w13230 {
              tunnel: [u16 0 ("Starting Address") u16 1184 ("Starting Address") u16 1185 ("Starting Address") u16 1186 ("Starting Address") u16 1187 ("Starting Address")] -> w13239
              tunnel: [u16 0 ("Ao_1_3") "Ch3_Ao_1_0 3" "Ch3_Ao_1_1 3" "Ch3_Ao_1_2 3" w13250] -> w13229
              frame #0 {
              }
              frame #1 {
              }
              frame #2 {
              }
              frame #3 {
              }
              frame #4 {
                n8419 = flat-sequence {
                  frame #0 {
                    n8420 = Wait (ms)(milliseconds to wait=u32 100) -> ()  [unwired: 1 out]
                  }
                  frame #1 {
                    n8421 = local write "Mfc2_Ar _3_4_set"(FALSE ("Mfc2_Ar _set")) -> ()
                  }
                }
                n8422 = Divide(x=2048.0, y=200.0) -> (x/y=w13251:dbl)
                n8423 = Multiply(x="Ar_sccm3_4", y=w13251) -> (x*y=w13250:dbl)
              }
            }
            n8424 = Build Array(w13229) -> (w13228:dbl[])
            n8425 = call-poly <vilib>:"MB Serial Master Query (poly).vi"("VISA resource name"=w13227, "Starting Address"=w13239, "Registers"=w13228, "error in"=w13226, "Serial Parameters"=T39 {"Mode"=enum."RTU", "Slave Address"=6}) -> ("VISA resource name out"=w13238:refnum<visa-resource-name>, "error out"=w13237:errorcluster)  [unwired: 1 in, 12 out]
          }
          frame #9 {
            n8426 = Wait (ms)(milliseconds to wait=w13257) -> ()  [unwired: 1 out]
          }
        }
      }
      frame #1 {
        n8427 = local read "Fail_moxa3_digital2"() -> (w13261:bool)
        n8428 = local read "Fail_moxa3_digital3"() -> (w13260:bool)
        n8429 = local read "Fail_moxa3_digital4"() -> (w13259:bool)
        n8430 = local read "Fail_moxa3_digital1"() -> (w13258:bool)
        n8431 = case shown="True" w13258 {
          frame #0 {
            w13329 = TRUE ("Mp_fail(ch3)")
            n8432 = local write "Ch3_Mp_fail"(w13329) -> ()
            n8433 = local write "Ch3_Tp_bv_fail"(w13329) -> ()
            n8434 = local write "Ch3_Bg_bv_fail"(w13329) -> ()
            n8435 = local write "Ch3_Ch_vbv_fail"(w13329) -> ()
            n8436 = local write "ch3_atm_fail_top"(w13329) -> ()
            n8437 = local write "ch3_bg_bv_fail_top"(w13329) -> ()
            n8438 = local write "ch3_cc_fail_top"(w13329) -> ()
            n8439 = local write "Ch3_Ch_vbv_fail"(w13329) -> ()
            n8440 = local write "Ch3_Ch_atm_fail"(w13329) -> ()
            n8441 = local write "Ch3_Pl_vbv_fail"(w13329) -> ()
            n8442 = local write "Ch3_Ch_cc_fail"(w13329) -> ()
            n8443 = local write "Ch3_Pl_atm_fail"(w13329) -> ()
          }
          frame #1 {
            n8444 = local read "Ch3_Mp_do"() -> (w13346:bool)
            n8445 = local read "Ch3_Mp_di"() -> (w13347:bool)
            n8446 = Exclusive Or(1:w13346, 2:w13347) -> (0:w13363:bool)
            n8447 = feedback #266() -> (w13364:bool)  [unwired: 1 in]
            n8448 = case shown="True" w13363 {
              tunnel: [TRUE FALSE] -> w13365
              tunnel: w13364 -> [_ w13406]
              tunnel: [FALSE w13403] -> w13345
              frame #0 {
              }
              frame #1 {
                n8449 = call "Elapsed Time113"("Reset"=w13406) -> ("Elapsed Time (s)"=w13405:dbl)  [unwired: 11 in, 7 out]
                n8450 = Greater?(x=w13405, y=5.0) -> (0:w13403:bool)
              }
            }
            n8451 = local write "Ch3_Mp_fail"(w13345) -> ()
            n8452 = local read "Ch3_Tp_bv_do"() -> (w13343:bool)
            n8453 = local read "Ch3_Tp_bv_di"() -> (w13344:bool)
            n8454 = Exclusive Or(1:w13343, 2:w13344) -> (0:w13362:bool)
            n8455 = feedback #267() -> (w13361:bool)  [unwired: 1 in]
            n8456 = case shown="True" w13362 {
              tunnel: [TRUE FALSE] -> w13360
              tunnel: w13361 -> [_ w13399]
              tunnel: [FALSE w13396] -> w13342
              frame #0 {
              }
              frame #1 {
                n8457 = call "Elapsed Time114"("Reset"=w13399) -> ("Elapsed Time (s)"=w13398:dbl)  [unwired: 11 in, 7 out]
                n8458 = Greater?(x=w13398, y=5.0) -> (0:w13396:bool)
              }
            }
            n8459 = local write "Ch3_Tp_bv_fail"(w13342) -> ()
            n8460 = local read "Ch3_Bg_bv_di"() -> (w13341:bool)
            n8461 = local read "Ch3_Bg_bv_do"() -> (w13340:bool)
            n8462 = Exclusive Or(1:w13340, 2:w13341) -> (0:w13357:bool)
            n8463 = feedback #268() -> (w13358:bool)  [unwired: 1 in]
            n8464 = case shown="True" w13357 {
              tunnel: [TRUE FALSE] -> w13359
              tunnel: w13358 -> [_ w13392]
              tunnel: [FALSE w13389] -> w13332
              frame #0 {
              }
              frame #1 {
                n8465 = call "Elapsed Time115"("Reset"=w13392) -> ("Elapsed Time (s)"=w13391:dbl)  [unwired: 11 in, 7 out]
                n8466 = Greater?(x=w13391, y=5.0) -> (0:w13389:bool)
              }
            }
            n8467 = local write "Ch3_Bg_bv_fail"(w13332) -> ()
            n8468 = local write "ch3_bg_bv_fail_top"(w13332) -> ()
            n8469 = local read "Ch3_Ch_vbv_do"() -> (w13339:bool)
            n8470 = local read "Ch3_Ch_vbv_di"() -> (w13333:bool)
            n8471 = Exclusive Or(1:w13339, 2:w13333) -> (0:w13356:bool)
            n8472 = feedback #269() -> (w13355:bool)  [unwired: 1 in]
            n8473 = case shown="True" w13356 {
              tunnel: [TRUE FALSE] -> w13354
              tunnel: w13355 -> [_ w13385]
              tunnel: [FALSE w13382] -> w13331
              frame #0 {
              }
              frame #1 {
                n8474 = call "Elapsed Time116"("Reset"=w13385) -> ("Elapsed Time (s)"=w13384:dbl)  [unwired: 11 in, 7 out]
                n8475 = Greater?(x=w13384, y=5.0) -> (0:w13382:bool)
              }
            }
            n8476 = local write "Ch3_Ch_vbv_fail"(w13331) -> ()
            n8477 = local read "Ch3_Pl_vbv_do"() -> (w13336:bool)
            n8478 = local read "Ch3_Pl_vbv_di"() -> (w13337:bool)
            n8479 = Exclusive Or(1:w13336, 2:w13337) -> (0:w13353:bool)
            n8480 = feedback #270() -> (w13352:bool)  [unwired: 1 in]
            n8481 = case shown="True" w13353 {
              tunnel: [TRUE FALSE] -> w13351
              tunnel: w13352 -> [_ w13378]
              tunnel: [FALSE w13375] -> w13338
              frame #0 {
              }
              frame #1 {
                n8482 = call "Elapsed Time118"("Reset"=w13378) -> ("Elapsed Time (s)"=w13377:dbl)  [unwired: 11 in, 7 out]
                n8483 = Greater?(x=w13377, y=5.0) -> (0:w13375:bool)
              }
            }
            n8484 = local read "Ch3_Cc_on_off_di"() -> (w13335:bool)
            n8485 = local write "Ch3_Pl_vbv_fail"(w13338) -> ()
            n8486 = local read "Ch3_Cc_on_off_do"() -> (w13334:bool)
            n8487 = feedback #271() -> (w13349:bool)  [unwired: 1 in]
            n8488 = Exclusive Or(1:w13334, 2:w13335) -> (0:w13350:bool)
            n8489 = case shown="True" w13350 {
              tunnel: [TRUE FALSE] -> w13348
              tunnel: w13349 -> [_ w13371]
              tunnel: [FALSE w13368] -> w13330
              frame #0 {